vi "FlexMag - 24-03-2023.vi"() -> ()   [LabVIEW 2018] (continued)
    n6375 = Match Pattern(string=w11431, regular expression="¢") -> (after substring=w11429:string)  [unwired: 4 out]
    n6376 = String Length(string=w11429) -> (length=w11433:i32)
    n6377 = String Subset(string=w11429, length (rest)=1 ("length (rest)")) -> (substring=w11427:string)  [unwired: 1 out]
    n6378 = String To Byte Array(string=w11427) -> (unsigned byte array=w11426:u8[])
    n6379 = Not Equal To 0?(x=w11433) -> (x != 0?=w11432:bool)
    n6380 = Index Array(array=w11426, index=0) -> (element=w11424:u8)
    n6381 = String To Byte Array(string=w11401) -> (unsigned byte array=w11406:u8[])
    n6382 = Number To Boolean Array(number=w11424) -> (Boolean array=w11423:bool[])
    n6383 = case shown="True" w11432 {
      tunnel: [w11788 w11792] -> w11374
      tunnel: [w11787 w11791] -> w11373
      tunnel: w11421 -> [w11788 w11790]
      tunnel: w11420 -> [w11787 w11789]
      frame False {
      }
      frame True {
        n6384 = VISA Write(VISA resource name=w11790, write buffer="\u0006", error in (no error)=w11789) -> (VISA resource name out=w11792:refnum<visa-resource-name>, error out=w11791:errorcluster)  [unwired: 1 out]
      }
    }
    n6385 = for {
      tunnel: w11406 -> [w11776] mode=indexing
      shift-right: [w11774] -> w11404
      shift-left: 0 -> [w11775]
      n6386 = Exclusive Or(1:w11775, 2:w11776) -> (0:w11774:i32)
    }
    n6387 = Index Array(array=w11423, index=6) -> (element=→"RF 1 On":bool)
    n6388 = Build Array(w11404) -> (w11403:i32[])
    n6389 = Byte Array To String(unsigned byte array=w11403) -> (string=w11402:string)
    n6390 = Concatenate Strings(w11401, w11402) -> (w11400:string)
    n6391 = VISA Write(VISA resource name=w11374, write buffer=w11400, error in (no error)=w11373) -> (VISA resource name out=w11416:refnum<visa-resource-name>, error out=w11415:errorcluster)  [unwired: 1 out]
    n6392 = stacked-sequence {
      tunnel: [w11786] -> w11412
      tunnel: w11416 -> [w11786]
      tunnel: [w11785] -> w11411
      tunnel: w11415 -> [w11785]
      frame #0 {
        n6393 = Wait Until Next ms Multiple(millisecond multiple=u32 40) -> ()  [unwired: 1 out]
      }
    }
    n6394 = property class="Instr"(reference=w11412, error in=w11411) -> (reference out=w11418:refnum<visa-resource-name>, error out=w11417:errorcluster, "Serial Settings:Number of Bytes at Serial Port"=w11376:u32)
    n6395 = VISA Read(VISA resource name=w11418, byte count=w11376, error in (no error)=w11417) -> (VISA resource name out=w11410:refnum<visa-resource-name>, read buffer=w11413:string, error out=w11409:errorcluster)  [unwired: 1 out]
    n6396 = Match Pattern(string=w11413, regular expression="—") -> (after substring=w11407:string)  [unwired: 4 out]
    n6397 = String Length(string=w11407) -> (length=w11408:i32)
    n6398 = String To Byte Array(string=w11407) -> (unsigned byte array=w11379:u8[])
    n6399 = Not Equal To 0?(x=w11408) -> (x != 0?=w11375:bool)
    n6400 = Index Array(array=w11379, index=1) -> (element=w11395:u8)
    n6401 = Index Array(array=w11379, index=0) -> (element=w11392:u8)
    n6402 = Index Array(array=w11379, index=3) -> (element=w11390:u8)
    n6403 = Index Array(array=w11379, index=2) -> (element=w11389:u8)
    n6404 = To Unsigned Long Integer(number=w11395) -> (unsigned 32bit integer=w11394:u32)
    n6405 = To Unsigned Long Integer(number=w11392) -> (unsigned 32bit integer=w11391:u32)
    n6406 = To Unsigned Long Integer(number=w11390) -> (unsigned 32bit integer=w11387:u32)
    n6407 = To Unsigned Long Integer(number=w11389) -> (unsigned 32bit integer=w11388:u32)
    n6408 = case shown="True" w11375 {
      tunnel: w11410 -> [w11778 w11782]
      tunnel: w11409 -> [w11777 w11781]
      tunnel: [w11778 w11780] -> w11367
      tunnel: [w11777 w11779] -> w11366
      frame False {
      }
      frame True {
        n6409 = VISA Write(VISA resource name=w11782, write buffer="\u0006", error in (no error)=w11781) -> (VISA resource name out=w11780:refnum<visa-resource-name>, error out=w11779:errorcluster)  [unwired: 1 out]
      }
    }
    n6410 = local read "Forward Power"() -> (w11362:u32)
    n6411 = local read "Reflected Power"() -> (w11361:u32)
    n6412 = Multiply(x=w11394, y=256) -> (x*y=w11397:u32)
    n6413 = Multiply(x=256, y=w11387) -> (x*y=w11385:u32)
    n6414 = Add(x=w11397, y=w11391) -> (x+y=w11380:u32)
    n6415 = Add(x=w11385, y=w11388) -> (x+y=w11381:u32)
    n6416 = Subtract(x=w11362, y=w11361) -> (x-y=→"RF Net Power :":u32)
    n6417 = Divide(x=w11380, y=u32 10) -> (x/y=w11378:dbl)
    n6418 = Divide(x=w11381, y=u32 10) -> (x/y=w11377:dbl)
    n6419 = case shown="True" w11375 {
      tunnel: w11378 -> [_ w11773]
      tunnel: w11377 -> [_ w11772]
      frame False {
      }
      frame True {
        "Ramp Up Left Time:" <- w11773
        "Ramp Down Left Time:" <- w11772
      }
    }
    n6420 = VISA Write(VISA resource name=w11367, write buffer="\bキ", error in (no error)=w11366) -> (VISA resource name out=w11689:refnum<visa-resource-name>, error out=w11687:errorcluster)  [unwired: 1 out]
    n6421 = stacked-sequence {
      tunnel: [w11887] -> w11690
      tunnel: w11689 -> [w11887]
      tunnel: [w11886] -> w11688
      tunnel: w11687 -> [w11886]
      frame #0 {
        n6422 = Wait Until Next ms Multiple(millisecond multiple=u32 40) -> ()  [unwired: 1 out]
      }
    }
    n6423 = property class="Instr"(reference=w11690, error in=w11688) -> (reference out=w11705:refnum<visa-resource-name>, error out=w11704:errorcluster, "Serial Settings:Number of Bytes at Serial Port"=w11706:u32)
    n6424 = VISA Read(VISA resource name=w11705, byte count=w11706, error in (no error)=w11704) -> (VISA resource name out=w11686:refnum<visa-resource-name>, read buffer=w11691:string, error out=w11685:errorcluster)  [unwired: 1 out]
    n6425 = Match Pattern(string=w11691, regular expression="¥") -> (after substring=w11683:string)  [unwired: 4 out]
    n6426 = String Length(string=w11683) -> (length=w11684:i32)
    n6427 = String Subset(string=w11683, length (rest)=2 ("length (rest)")) -> (substring=w11701:string)  [unwired: 1 out]
    n6428 = Not Equal To 0?(x=w11684) -> (x != 0?=w11458:bool)
    n6429 = String To Byte Array(string=w11701) -> (unsigned byte array=w11699:u8[])
    n6430 = case shown="True" w11458 {
      tunnel: w11686 -> [w11880 w11884]
      tunnel: w11685 -> [w11879 w11883]
      tunnel: [w11880 w11882] -> w11661
      tunnel: [w11879 w11881] -> w11660
      frame False {
      }
      frame True {
        n6431 = VISA Write(VISA resource name=w11884, write buffer="\u0006", error in (no error)=w11883) -> (VISA resource name out=w11882:refnum<visa-resource-name>, error out=w11881:errorcluster)  [unwired: 1 out]
      }
    }
    n6432 = Index Array(array=w11699, index=1) -> (element=w11696:u8)
    n6433 = Index Array(array=w11699, index=0) -> (element=w11693:u8)
    n6434 = To Unsigned Long Integer(number=w11696) -> (unsigned 32bit integer=w11695:u32)
    n6435 = To Unsigned Long Integer(number=w11693) -> (unsigned 32bit integer=w11692:u32)
    n6436 = Multiply(x=256, y=w11695) -> (x*y=w11694:u32)
    n6437 = Add(x=w11694, y=w11692) -> (x+y=w11507:u32)
    n6438 = case shown="True" w11458 {
      tunnel: w11507 -> [_ w11817]
      frame False {
      }
      frame True {
        "Forward Power" <- w11817
      }
    }
    n6439 = VISA Write(VISA resource name=w11661, write buffer="\b¨ ", error in (no error)=w11660) -> (VISA resource name out=w11666:refnum<visa-resource-name>, error out=w11665:errorcluster)  [unwired: 1 out]
    n6440 = stacked-sequence {
      tunnel: [w11878] -> w11664
      tunnel: w11666 -> [w11878]
      tunnel: [w11877] -> w11663
      tunnel: w11665 -> [w11877]
      frame #0 {
        n6441 = Wait Until Next ms Multiple(millisecond multiple=u32 40) -> ()  [unwired: 1 out]
      }
    }
    n6442 = property class="Instr"(reference=w11664, error in=w11663) -> (reference out=w11682:refnum<visa-resource-name>, error out=w11680:errorcluster, "Serial Settings:Number of Bytes at Serial Port"=w11681:u32)
    n6443 = VISA Read(VISA resource name=w11682, byte count=w11681, error in (no error)=w11680) -> (VISA resource name out=w11659:refnum<visa-resource-name>, read buffer=w11679:string, error out=w11658:errorcluster)  [unwired: 1 out]
    n6444 = Match Pattern(string=w11679, regular expression="¨") -> (after substring=w11657:string)  [unwired: 4 out]
    n6445 = String Length(string=w11657) -> (length=w11656:i32)
    n6446 = String Subset(string=w11657, length (rest)=2 ("length (rest)")) -> (substring=w11676:string)  [unwired: 1 out]
    n6447 = Not Equal To 0?(x=w11656) -> (x != 0?=w11457:bool)
    n6448 = String To Byte Array(string=w11676) -> (unsigned byte array=w11674:u8[])
    n6449 = case shown="True" w11457 {
      tunnel: w11659 -> [w11870 w11874]
      tunnel: w11658 -> [w11869 w11873]
      tunnel: [w11870 w11872] -> w11620
      tunnel: [w11869 w11871] -> w11613
      frame False {
      }
      frame True {
        n6450 = VISA Write(VISA resource name=w11874, write buffer="\u0006", error in (no error)=w11873) -> (VISA resource name out=w11872:refnum<visa-resource-name>, error out=w11871:errorcluster)  [unwired: 1 out]
      }
    }
    n6451 = Index Array(array=w11674, index=1) -> (element=w11669:u8)
    n6452 = Index Array(array=w11674, index=0) -> (element=w11670:u8)
    n6453 = To Unsigned Long Integer(number=w11669) -> (unsigned 32bit integer=w11672:u32)
    n6454 = To Unsigned Long Integer(number=w11670) -> (unsigned 32bit integer=w11667:u32)
    n6455 = Multiply(x=256, y=w11672) -> (x*y=w11668:u32)
    n6456 = Add(x=w11668, y=w11667) -> (x+y=w11506:u32)
    n6457 = case shown="True" w11457 {
      tunnel: w11506 -> [_ w11816]
      frame False {
      }
      frame True {
        "RF Bias:" <- w11816
      }
    }
    n6458 = VISA Write(VISA resource name=w11620, write buffer="\b¯§", error in (no error)=w11613) -> (VISA resource name out=w11652:refnum<visa-resource-name>, error out=w11651:errorcluster)  [unwired: 1 out]
    n6459 = stacked-sequence {
      tunnel: [w11868] -> w11625
      tunnel: w11652 -> [w11868]
      tunnel: [w11867] -> w11624
      tunnel: w11651 -> [w11867]
      frame #0 {
        n6460 = Wait Until Next ms Multiple(millisecond multiple=u32 40) -> ()  [unwired: 1 out]
      }
    }
    n6461 = property class="Instr"(reference=w11625, error in=w11624) -> (reference out=w11654:refnum<visa-resource-name>, error out=w11653:errorcluster, "Serial Settings:Number of Bytes at Serial Port"=w11655:u32)
    n6462 = VISA Read(VISA resource name=w11654, byte count=w11655, error in (no error)=w11653) -> (VISA resource name out=w11619:refnum<visa-resource-name>, read buffer=w11626:string, error out=w11618:errorcluster)  [unwired: 1 out]
    n6463 = Match Pattern(string=w11626, regular expression="¯") -> (after substring=w11616:string)  [unwired: 4 out]
    n6464 = String Length(string=w11616) -> (length=w11617:i32)
    n6465 = String Subset(string=w11616, length (rest)=2 ("length (rest)")) -> (substring=w11643:string)  [unwired: 1 out]
    n6466 = String Subset(string=w11616, offset (0)=2, length (rest)=2 ("length (rest)")) -> (substring=w11638:string)
    n6467 = Not Equal To 0?(x=w11617) -> (x != 0?=w11456:bool)
    n6468 = String To Byte Array(string=w11643) -> (unsigned byte array=w11646:u8[])
    n6469 = String To Byte Array(string=w11638) -> (unsigned byte array=w11640:u8[])
    n6470 = case shown="True" w11456 {
      tunnel: [w11860 w11864] -> w11594
      tunnel: [w11859 w11863] -> w11593
      tunnel: w11619 -> [w11860 w11862]
      tunnel: w11618 -> [w11859 w11861]
      frame False {
      }
      frame True {
        n6471 = VISA Write(VISA resource name=w11862, write buffer="\u0006", error in (no error)=w11861) -> (VISA resource name out=w11864:refnum<visa-resource-name>, error out=w11863:errorcluster)  [unwired: 1 out]
      }
    }
    n6472 = Index Array(array=w11646, index=1) -> (element=w11637:u8)
    n6473 = Index Array(array=w11646, index=0) -> (element=w11634:u8)
    n6474 = Index Array(array=w11640, index=1) -> (element=w11632:u8)
    n6475 = Index Array(array=w11640, index=0) -> (element=w11631:u8)
    n6476 = To Unsigned Long Integer(number=w11637) -> (unsigned 32bit integer=w11636:u32)
    n6477 = To Unsigned Long Integer(number=w11634) -> (unsigned 32bit integer=w11633:u32)
    n6478 = To Unsigned Long Integer(number=w11632) -> (unsigned 32bit integer=w11629:u32)
    n6479 = To Unsigned Long Integer(number=w11631) -> (unsigned 32bit integer=w11630:u32)
    n6480 = Multiply(x=w11636, y=256) -> (x*y=w11644:u32)
    n6481 = Multiply(x=256, y=w11629) -> (x*y=w11627:u32)
    n6482 = Add(x=w11644, y=w11633) -> (x+y=w11614:u32)
    n6483 = Add(x=w11627, y=w11630) -> (x+y=w11615:u32)
    n6484 = case shown="True" w11456 {
      tunnel: u32 10 ("y") -> [_ w11815]
      tunnel: u32 10 ("y") -> [_ w11814]
      tunnel: w11615 -> [_ w11813]
      tunnel: w11614 -> [_ w11812]
      frame False {
      }
      frame True {
        n6485 = Divide(x=w11812, y=w11815) -> (x/y=→"CL Position:":dbl)
        n6486 = Divide(x=w11813, y=w11814) -> (x/y=→"CT Position:":dbl)
      }
    }
    n6487 = VISA Write(VISA resource name=w11594, write buffer="\bš’", error in (no error)=w11593) -> (VISA resource name out=w11609:refnum<visa-resource-name>, error out=w11608:errorcluster)  [unwired: 1 out]
    n6488 = stacked-sequence {
      tunnel: [w11858] -> w11596
      tunnel: w11609 -> [w11858]
      tunnel: [w11857] -> w11595
      tunnel: w11608 -> [w11857]
      frame #0 {
        n6489 = Wait Until Next ms Multiple(millisecond multiple=u32 40) -> ()  [unwired: 1 out]
      }
    }
    n6490 = property class="Instr"(reference=w11596, error in=w11595) -> (reference out=w11611:refnum<visa-resource-name>, error out=w11610:errorcluster, "Serial Settings:Number of Bytes at Serial Port"=w11612:u32)
    n6491 = VISA Read(VISA resource name=w11611, byte count=w11612, error in (no error)=w11610) -> (VISA resource name out=w11592:refnum<visa-resource-name>, read buffer=w11597:string, error out=w11591:errorcluster)  [unwired: 1 out]
    n6492 = Match Pattern(string=w11597, regular expression="\u0006\tš") -> (after substring=w11589:string)  [unwired: 4 out]
    n6493 = String Length(string=w11589) -> (length=w11590:i32)
    n6494 = String Subset(string=w11589, length (rest)=1 ("length (rest)")) -> (substring=w11598:string)  [unwired: 1 out]
    n6495 = Not Equal To 0?(x=w11590) -> (x != 0?=w11455:bool)
    n6496 = Match True/False String(2:"" ("false string"), 3:"\u0006" ("true string"), 4:w11598) -> (0:w11505:bool)  [unwired: 1 out]
    n6497 = Match True/False String(2:"" ("false string"), 3:"\b" ("true string"), 4:w11598) -> (0:w11504:bool)  [unwired: 1 out]
    n6498 = Match True/False String(2:"" ("false string"), 3:"\u0007" ("true string"), 4:w11598) -> (0:w11503:bool)  [unwired: 1 out]
    n6499 = case shown="True" w11455 {
      tunnel: [w11850 w11854] -> w11568
      tunnel: [w11849 w11851] -> w11567
      tunnel: w11592 -> [w11850 w11853]
      tunnel: w11591 -> [w11849 w11852]
      frame False {
      }
      frame True {
        n6500 = VISA Write(VISA resource name=w11853, write buffer="\u0006", error in (no error)=w11852) -> (VISA resource name out=w11854:refnum<visa-resource-name>, error out=w11851:errorcluster)  [unwired: 1 out]
      }
    }
    n6501 = case shown="True" w11455 {
      tunnel: w11505 -> [_ w11809]
      tunnel: w11504 -> [_ w11808]
      tunnel: w11503 -> [_ w11807]
      frame False {
      }
      frame True {
        "FORWARD   REGULATION" <- w11809
        "LOAD  REGULATION" <- w11807
        "DC BIAS REGULATION" <- w11808
      }
    }
    n6502 = VISA Write(VISA resource name=w11568, write buffer="\b惫", error in (no error)=w11567) -> (VISA resource name out=w11582:refnum<visa-resource-name>, error out=w11581:errorcluster)  [unwired: 1 out]
    n6503 = stacked-sequence {
      tunnel: [w11848] -> w11570
      tunnel: w11582 -> [w11848]
      tunnel: [w11847] -> w11569
      tunnel: w11581 -> [w11847]
      frame #0 {
        n6504 = Wait Until Next ms Multiple(millisecond multiple=u32 40) -> ()  [unwired: 1 out]
      }
    }
    n6505 = property class="Instr"(reference=w11570, error in=w11569) -> (reference out=w11584:refnum<visa-resource-name>, error out=w11583:errorcluster, "Serial Settings:Number of Bytes at Serial Port"=w11585:u32)
    n6506 = VISA Read(VISA resource name=w11584, byte count=w11585, error in (no error)=w11583) -> (VISA resource name out=w11566:refnum<visa-resource-name>, read buffer=w11571:string, error out=w11565:errorcluster)  [unwired: 1 out]
    n6507 = Match Pattern(string=w11571, regular expression="±") -> (after substring=w11563:string)  [unwired: 4 out]
    n6508 = String Subset(string=w11563) -> (substring=w11572:string)  [unwired: 2 out]
    n6509 = String Length(string=w11563) -> (length=w11564:i32)
    n6510 = Not Equal To 0?(x=w11564) -> (x != 0?=w11454:bool)
    n6511 = Match True/False String(2:"" ("false string"), 3:"\u0002" ("true string"), 4:w11572) -> (0:w11502:bool)  [unwired: 1 out]
    n6512 = Match True/False String(2:"" ("false string"), 3:"\u0000" ("true string"), 4:w11572) -> (0:w11501:bool)  [unwired: 1 out]
    n6513 = Match True/False String(2:"" ("false string"), 3:"\u0001" ("true string"), 4:w11572) -> (0:w11500:bool)  [unwired: 1 out]
    n6514 = case shown="True" w11454 {
      tunnel: [w11840 w11842] -> w11550
      tunnel: [w11839 w11841] -> w11549
      tunnel: w11566 -> [w11840 w11844]
      tunnel: w11565 -> [w11839 w11843]
      frame False {
      }
      frame True {
        n6515 = VISA Write(VISA resource name=w11844, write buffer="\u0006", error in (no error)=w11843) -> (VISA resource name out=w11842:refnum<visa-resource-name>, error out=w11841:errorcluster)  [unwired: 1 out]
      }
    }
    n6516 = case shown="True" w11454 {
      tunnel: w11502 -> [_ w11806]
      tunnel: w11501 -> [_ w11805]
      tunnel: w11500 -> [_ w11803]
      frame False {
      }
      frame True {
        n6517 = Not(x=w11805) -> (.not. x?=w11804:bool)
        n6518 = And(x=w11804, y=w11803) -> (x .and. y?=→"Pulsing ON/OFF :":bool)
        "INTERNAL PULSING" <- w11803
        "PULSING OFF" <- w11805
        "EXTERNAL PULSING" <- w11806
      }
    }
    n6519 = VISA Write(VISA resource name=w11550, write buffer="\b奶", error in (no error)=w11549) -> (VISA resource name out=w11559:refnum<visa-resource-name>, error out=w11558:errorcluster)  [unwired: 1 out]
    n6520 = stacked-sequence {
      tunnel: [w11838] -> w11552
      tunnel: w11559 -> [w11838]
      tunnel: [w11837] -> w11551
      tunnel: w11558 -> [w11837]
      frame #0 {
        n6521 = Wait Until Next ms Multiple(millisecond multiple=u32 40) -> ()  [unwired: 1 out]
      }
    }
    n6522 = property class="Instr"(reference=w11552, error in=w11551) -> (reference out=w11561:refnum<visa-resource-name>, error out=w11560:errorcluster, "Serial Settings:Number of Bytes at Serial Port"=w11562:u32)
    n6523 = VISA Read(VISA resource name=w11561, byte count=w11562, error in (no error)=w11560) -> (VISA resource name out=w11548:refnum<visa-resource-name>, read buffer=w11553:string, error out=w11547:errorcluster)  [unwired: 1 out]
    n6524 = Match Pattern(string=w11553, regular expression="Ä") -> (after substring=w11545:string)  [unwired: 4 out]
    n6525 = String To Byte Array(string=w11545) -> (unsigned byte array=w11555:u8[])
    n6526 = String Length(string=w11545) -> (length=w11453:i32)
    n6527 = Not Equal To 0?(x=w11453) -> (x != 0?=w11546:bool)
    n6528 = Index Array(array=w11555, index=0) -> (element=w11499:u8)
    n6529 = case shown="1" w11453 {
      tunnel: w11499 -> [_ w11801]
      frame 0, Default {
      }
      frame 1 {
        "duty cycle" <- w11801
      }
    }
    n6530 = case shown="True" w11546 {
      tunnel: [w11830 w11832] -> w11515
      tunnel: [w11829 w11831] -> w11514
      tunnel: w11548 -> [w11830 w11834]
      tunnel: w11547 -> [w11829 w11833]
      frame False {
      }
      frame True {
        n6531 = VISA Write(VISA resource name=w11834, write buffer="\u0006", error in (no error)=w11833) -> (VISA resource name out=w11832:refnum<visa-resource-name>, error out=w11831:errorcluster)  [unwired: 1 out]
      }
    }
    n6532 = VISA Write(VISA resource name=w11515, write buffer="\b辽", error in (no error)=w11514) -> (VISA resource name out=w11541:refnum<visa-resource-name>, error out=w11540:errorcluster)  [unwired: 1 out]
    n6533 = stacked-sequence {
      tunnel: [w11828] -> w11517
      tunnel: w11541 -> [w11828]
      tunnel: [w11827] -> w11516
      tunnel: w11540 -> [w11827]
      frame #0 {
        n6534 = Wait Until Next ms Multiple(millisecond multiple=u32 40) -> ()  [unwired: 1 out]
      }
    }
    n6535 = property class="Instr"(reference=w11517, error in=w11516) -> (reference out=w11543:refnum<visa-resource-name>, error out=w11542:errorcluster, "Serial Settings:Number of Bytes at Serial Port"=w11544:u32)
    n6536 = VISA Read(VISA resource name=w11543, byte count=w11544, error in (no error)=w11542) -> (VISA resource name out=w11513:refnum<visa-resource-name>, read buffer=w11518:string, error out=w11512:errorcluster)  [unwired: 1 out]
    n6537 = Match Pattern(string=w11518, regular expression="Á") -> (after substring=w11508:string)  [unwired: 4 out]
    n6538 = String To Byte Array(string=w11508) -> (unsigned byte array=w11531:u8[])
    n6539 = String Length(string=w11508) -> (length=w11452:i32)
    n6540 = Index Array(array=w11531, index=3) -> (element=w11523:u8)
    n6541 = Index Array(array=w11531, index=2) -> (element=w11526:u8)
    n6542 = Index Array(array=w11531, index=1) -> (element=w11535:u8)
    n6543 = Index Array(array=w11531, index=0) -> (element=w11533:u8)
    n6544 = Not Equal To 0?(x=w11452) -> (x != 0?=w11509:bool)
    n6545 = To Unsigned Long Integer(number=w11523) -> (unsigned 32bit integer=w11525:u32)
    n6546 = To Unsigned Long Integer(number=w11526) -> (unsigned 32bit integer=w11528:u32)
    n6547 = To Unsigned Long Integer(number=w11535) -> (unsigned 32bit integer=w11534:u32)
    n6548 = To Unsigned Long Integer(number=w11533) -> (unsigned 32bit integer=w11519:u32)
    n6549 = case shown="True" w11509 {
      tunnel: [w11820 w11822] -> w11511
      tunnel: [w11819 w11821] -> w11510
      tunnel: w11513 -> [w11820 w11824]
      tunnel: w11512 -> [w11819 w11823]
      frame False {
      }
      frame True {
        n6550 = VISA Write(VISA resource name=w11824, write buffer="\u0006", error in (no error)=w11823) -> (VISA resource name out=w11822:refnum<visa-resource-name>, error out=w11821:errorcluster)  [unwired: 1 out]
      }
    }
    n6551 = Multiply(x=256, y=w11525) -> (x*y=w11522:u32)
    n6552 = Multiply(x=256, y=w11528) -> (x*y=w11521:u32)
    n6553 = Multiply(x=256, y=w11534) -> (x*y=w11520:u32)
    n6554 = Compound Arithmetic op=ADD(w11522, w11521, w11520, w11519) -> (w11498:u32)
    n6555 = case shown="1" w11452 {
      tunnel: w11498 -> [_ w11800]
      frame 0, Default {
      }
      frame 1 {
        "Frequency" <- w11800
      }
    }
  }
  n6556 = property on="Tab Pressure Graph" class="TabCtl (strict)"("Visible"=FALSE) -> ()  [unwired: 2 in, 2 out]
  n6557 = while {
    i -> [w12239]
    stop <- FALSE stop-if-true
    n6558 = Get Date/Time String(want seconds? (F)=TRUE) -> (time string=w12257:string)  [unwired: 2 in, 1 out]
    "time string" <- w12257
    n6559 = local read "hour s"() -> (w12248:string)
    n6560 = local read "min s"() -> (w12247:string)
    n6561 = local read "sec s"() -> (w12246:string)
    n6562 = Match Pattern(string=w12257, regular expression=":") -> (before substring=→"hour s":string, after substring=w12255:string)  [unwired: 1 in, 2 out]
    n6563 = Match Pattern(string=w12255, regular expression=":") -> (before substring=→"min s":string, after substring=w12251:string)  [unwired: 1 in, 2 out]
    n6564 = call <vilib>:"Space Constant.vi"() -> ("String"=w12250:string)
    n6565 = Multiply(x=1000, y="graph sec") -> (x*y=w12242:dbl)
    n6566 = Decimal String To Number(string=w12248) -> (number=→"hour":i32)  [unwired: 2 in, 1 out]
    n6567 = Decimal String To Number(string=w12247) -> (number=→"min":i32)  [unwired: 2 in, 1 out]
    n6568 = Decimal String To Number(string=w12246) -> (number=→"sec":i32)  [unwired: 2 in, 1 out]
    n6569 = Build Array(FALSE, "show pressure graphs", "hide pressure graphs") -> (w12263:bool[])
    n6570 = Wait Until Next ms Multiple(millisecond multiple=w12242) -> ()  [unwired: 1 out]
    n6571 = Match Pattern(string=w12251, regular expression=w12250) -> (before substring=→"sec s":string)  [unwired: 1 in, 3 out]
    n6572 = Boolean Array To Number(Boolean array=w12263) -> (number=w12264:u32)
    n6573 = Mantissa & Exponent(0:w12264) -> (2:w12259:dbl)  [unwired: 1 out]
    n6574 = case shown="0, Default" w12259 {
      frame 0, Default {
      }
      frame 1 {
        n6575 = property on="Tab Pressure Graph" class="TabCtl (strict)"("Visible"=TRUE) -> ()  [unwired: 2 in, 2 out]
      }
      frame 2 {
        n6576 = property on="Tab Pressure Graph" class="TabCtl (strict)"("Visible"=FALSE) -> ()  [unwired: 2 in, 2 out]
      }
    }
    n6577 = local read "CH4_CC_DI"() -> (w12235:bool)
    n6578 = local read "CH3_CC_DI"() -> (w12236:bool)
    n6579 = local read "CH2_CC_DI"() -> (w12237:bool)
    n6580 = local read "CH1_CC_DI"() -> (w12238:bool)
    n6581 = case shown="False" w12235 {
      tunnel: [w12266 w12267] -> w12232
      frame False {
        n6582 = local read "ch4 ch pg mbar"() -> (w12266:dbl)
      }
      frame True {
        n6583 = local read "ch4 cc mbar"() -> (w12267:dbl)
      }
    }
    "CH 4 Pressure" <- w12232
    n6584 = case shown="False" w12236 {
      tunnel: [w12268 w12269] -> w12231
      frame False {
        n6585 = local read "ch3 ch pg mbar"() -> (w12268:dbl)
      }
      frame True {
        n6586 = local read "ch3 cc mbar"() -> (w12269:dbl)
      }
    }
    "CH 3 Pressure" <- w12231
    n6587 = case shown="False" w12237 {
      tunnel: [w12270 w12271] -> w12233
      frame False {
        n6588 = local read "ch2 ch pg mbar"() -> (w12270:dbl)
      }
      frame True {
        n6589 = local read "ch2 cc mbar"() -> (w12271:dbl)
      }
    }
    "CH 2 Pressure" <- w12233
    n6590 = case shown="False" w12238 {
      tunnel: [w12272 w12273] -> w12234
      frame False {
        n6591 = local read "ch1 ch pg mbar"() -> (w12272:dbl)
      }
      frame True {
        n6592 = local read "ch1 cc mbar"() -> (w12273:dbl)
      }
    }
    "CH 1 Pressure" <- w12234
    "iteration for graph" <- w12239
  }
  n6593 = while {
    i -> [w12277]
    stop <- FALSE stop-if-true
    n6594 = Greater?(x=w12277, y=u32 10 ("millisecond multiple")) -> (0:w12276:bool)
    n6595 = Wait Until Next ms Multiple(millisecond multiple=u32 1000) -> ()  [unwired: 1 out]
    n6596 = case shown="True" w12276 {
      frame False {
        n6597 = local read "ch2 ch pg torr"() -> (w12301:dbl)
        n6598 = local read "ch1 ch pg torr"() -> (w12304:dbl)
        n6599 = local read "ch3 ch pg torr"() -> (w12300:dbl)
        n6600 = local read "ch4 ch pg torr"() -> (w12293:dbl)
        n6601 = local read "ch2 ch pg torr"() -> (w12297:dbl)
        n6602 = local read "ch3 ch pg torr"() -> (w12296:dbl)
        n6603 = Less Or Equal?(x=w12301, y=50.0) -> (x <= y?=w12291:bool)
        n6604 = Less Or Equal?(x=w12304, y=50.0) -> (x <= y?=w12292:bool)
        n6605 = Less Or Equal?(x=w12300, y=50.0) -> (x <= y?=w12289:bool)
        n6606 = Less Or Equal?(x=w12293, y=50.0) -> (x <= y?=w12287:bool)
        n6607 = Less Or Equal?(x=w12297, y=50.0) -> (x <= y?=w12290:bool)
        n6608 = Less Or Equal?(x=w12296, y=50.0) -> (x <= y?=w12288:bool)
        n6609 = And(x=w12292, y=w12291) -> (x .and. y?=w12285:bool)
        n6610 = And(x=w12288, y=w12287) -> (x .and. y?=w12286:bool)
        n6611 = And(x=w12290, y=w12289) -> (x .and. y?=w12284:bool)
        n6612 = case shown="True" w12285 {
          tunnel: ["ATMOSPHERE" "VACUUM"] -> w12281
          frame False {
          }
          frame True {
          }
        }
        "ch1_2 vacuum level" <- w12281
        n6613 = case shown="True" w12284 {
          tunnel: ["ATMOSPHERE" "VACUUM"] -> w12283
          frame False {
          }
          frame True {
          }
        }
        "ch2_3 vacuum level" <- w12283
        n6614 = case shown="True" w12286 {
          tunnel: ["ATMOSPHERE" "VACUUM"] -> w12282
          frame False {
          }
          frame True {
          }
        }
        "ch3_4 vacuum level" <- w12282
      }
      frame True {
        n6615 = stacked-sequence {
          frame #0 {
            n6616 = local read "ch3_gv_bp_right_gui"() -> (w12334:bool)
            n6617 = local read "ch4_gv_bp_right_gui"() -> (w12324:bool)
            n6618 = local read "ch2_gv_bp_right_gui"() -> (w12344:bool)
            n6619 = local read "ch3_gv_bp_left_gui"() -> (w12325:bool)
            n6620 = local read "ch2_gv_bp_left_gui"() -> (w12335:bool)
            n6621 = local read "ch1_gv_bp_left_gui"() -> (w12345:bool)
            n6622 = feedback #181() -> (w12331:bool)  [unwired: 1 in]
            n6623 = feedback-in #181(w12334) -> ()
            n6624 = feedback #182() -> (w12328:bool)  [unwired: 1 in]
            n6625 = feedback-in #182(w12325) -> ()
            n6626 = feedback #183() -> (w12321:bool)  [unwired: 1 in]
            n6627 = feedback-in #183(w12324) -> ()
            n6628 = feedback #184() -> (w12338:bool)  [unwired: 1 in]
            n6629 = feedback-in #184(w12335) -> ()
            n6630 = feedback #185() -> (w12348:bool)  [unwired: 1 in]
            n6631 = feedback-in #185(w12345) -> ()
            n6632 = feedback #186() -> (w12341:bool)  [unwired: 1 in]
            n6633 = feedback-in #186(w12344) -> ()
            n6634 = Boolean To (0,1)(Boolean=w12334) -> (0, 1=w12330:i16)
            n6635 = Boolean To (0,1)(Boolean=w12325) -> (0, 1=w12329:i16)
            n6636 = Boolean To (0,1)(Boolean=w12324) -> (0, 1=w12320:i16)
            n6637 = Boolean To (0,1)(Boolean=w12335) -> (0, 1=w12339:i16)
            n6638 = Boolean To (0,1)(Boolean=w12331) -> (0, 1=w12332:i16)
            n6639 = Boolean To (0,1)(Boolean=w12328) -> (0, 1=w12327:i16)
            n6640 = Boolean To (0,1)(Boolean=w12321) -> (0, 1=w12322:i16)
            n6641 = Boolean To (0,1)(Boolean=w12345) -> (0, 1=w12349:i16)
            n6642 = Boolean To (0,1)(Boolean=w12344) -> (0, 1=w12340:i16)
            n6643 = Boolean To (0,1)(Boolean=w12338) -> (0, 1=w12337:i16)
            n6644 = Boolean To (0,1)(Boolean=w12348) -> (0, 1=w12347:i16)
            n6645 = Boolean To (0,1)(Boolean=w12341) -> (0, 1=w12342:i16)
            n6646 = Not Equal?(x=w12330, y=w12332) -> (x != y?=w12333:bool)
            n6647 = Not Equal?(x=w12329, y=w12327) -> (x != y?=w12326:bool)
            n6648 = Not Equal?(x=w12320, y=w12322) -> (x != y?=w12323:bool)
            n6649 = Not Equal?(x=w12339, y=w12337) -> (x != y?=w12336:bool)
            n6650 = Not Equal?(x=w12349, y=w12347) -> (x != y?=w12346:bool)
            n6651 = Not Equal?(x=w12340, y=w12342) -> (x != y?=w12343:bool)
            n6652 = case shown="True" w12333 {
              tunnel: w12334 -> [_ w12392]
              tunnel: [FALSE w12391] -> w12314
              frame False {
              }
              frame True {
                n6653 = case shown="True" w12392 {
                  tunnel: [FALSE TRUE] -> w12391
                  frame False {
                  }
                  frame True {
                  }
                }
              }
            }
            n6654 = case shown="True" w12326 {
              tunnel: w12325 -> [_ w12387]
              tunnel: [FALSE w12386] -> w12312
              frame False {
              }
              frame True {
                n6655 = case shown="True" w12387 {
                  tunnel: [FALSE TRUE] -> w12386
                  frame False {
                  }
                  frame True {
                  }
                }
              }
            }
            n6656 = case shown="True" w12323 {
              tunnel: w12324 -> [_ w12382]
              tunnel: [FALSE w12381] -> w12311
              frame False {
              }
              frame True {
                n6657 = case shown="True" w12382 {
                  tunnel: [FALSE TRUE] -> w12381
                  frame False {
                  }
                  frame True {
                  }
                }
              }
            }
            n6658 = case shown="True" w12336 {
              tunnel: w12335 -> [_ w12397]
              tunnel: [FALSE w12396] -> w12315
              frame False {
              }
              frame True {
                n6659 = case shown="True" w12397 {
                  tunnel: [FALSE TRUE] -> w12396
                  frame False {
                  }
                  frame True {
                  }
                }
              }
            }
            n6660 = case shown="True" w12346 {
              tunnel: w12345 -> [_ w12407]
              tunnel: [FALSE w12406] -> w12319
              frame False {
              }
              frame True {
                n6661 = case shown="True" w12407 {
                  tunnel: [FALSE TRUE] -> w12406
                  frame False {
                  }
                  frame True {
                  }
                }
              }
            }
            n6662 = case shown="True" w12343 {
              tunnel: w12344 -> [_ w12402]
              tunnel: [FALSE w12401] -> w12318
              frame False {
              }
              frame True {
                n6663 = case shown="True" w12402 {
                  tunnel: [FALSE TRUE] -> w12401
                  frame False {
                  }
                  frame True {
                  }
                }
              }
            }
            n6664 = Or(x=w12319, y=w12318) -> (x .or. y?=w12317:bool)
            n6665 = Or(x=w12315, y=w12314) -> (x .or. y?=w12316:bool)
            n6666 = Or(x=w12312, y=w12311) -> (x .or. y?=w12313:bool)
            n6667 = case shown="True" w12317 {
              frame False {
              }
              frame True {
                n6668 = local read "ch1 ch pg torr"() -> (w12377:dbl)
                n6669 = local read "ch2 ch pg torr"() -> (w12376:dbl)
                n6670 = Less?(x=w12377, y=0.5) -> (x < y?=w12373:bool)
                n6671 = Less?(x=w12376, y=0.5) -> (x < y?=w12372:bool)
                n6672 = And(x=w12373, y=w12372) -> (x .and. y?=w12370:bool)
                n6673 = case shown="False" w12370 {
                  tunnel: ["ATMOSPHERE" "VACUUM"] -> w12371
                  frame False {
                  }
                  frame True {
                  }
                }
                n6674 = local write "ch1_2 vacuum level"(w12371) -> ()
              }
            }
            n6675 = case shown="True" w12316 {
              frame False {
              }
              frame True {
                n6676 = local read "ch2 ch pg torr"() -> (w12367:dbl)
                n6677 = local read "ch3 ch pg torr"() -> (w12366:dbl)
                n6678 = Less?(x=w12367, y=0.5) -> (x < y?=w12363:bool)
                n6679 = Less?(x=w12366, y=0.5) -> (x < y?=w12362:bool)
                n6680 = And(x=w12363, y=w12362) -> (x .and. y?=w12361:bool)
                n6681 = case shown="True" w12361 {
                  tunnel: ["ATMOSPHERE" "VACUUM"] -> w12360
                  frame False {
                  }
                  frame True {
                  }
                }
                n6682 = local write "ch2_3 vacuum level"(w12360) -> ()
              }
            }
            n6683 = case shown="True" w12313 {
              frame False {
              }
              frame True {
                n6684 = local read "ch3 ch pg torr"() -> (w12357:dbl)
                n6685 = local read "ch4 ch pg torr"() -> (w12356:dbl)
                n6686 = Less?(x=w12357, y=0.5) -> (x < y?=w12353:bool)
                n6687 = Less?(x=w12356, y=0.5) -> (x < y?=w12352:bool)
                n6688 = And(x=w12353, y=w12352) -> (x .and. y?=w12351:bool)
                n6689 = case shown="False" w12351 {
                  tunnel: ["ATMOSPHERE" "VACUUM"] -> w12350
                  frame False {
                  }
                  frame True {
                  }
                }
                n6690 = local write "ch3_4 vacuum level"(w12350) -> ()
              }
            }
          }
          frame #1 {
            n6691 = local read "CH2_Trns_BP_Right_DI"() -> (w12414:bool)
            n6692 = local read "CH3_Trns_BP_Right_DI"() -> (w12413:bool)
            n6693 = local read "CH4_Trns_BP_Right_DI"() -> (w12410:bool)
            n6694 = local read "CH1_Trns_BP_Left_DI"() -> (w12415:bool)
            n6695 = local read "CH2_Trns_BP_Left_DI"() -> (w12412:bool)
            n6696 = local read "CH3_Trns_BP_Left_DI"() -> (w12411:bool)
            n6697 = case shown="True" w12415 {
              frame False {
              }
              frame True {
                n6698 = local read "ch1 ch pg torr"() -> (w12449:dbl)
                n6699 = Less?(x=w12449, y=0.5) -> (x < y?=w12446:bool)
                n6700 = case shown="True" w12446 {
                  tunnel: ["ATMOSPHERE" "VACUUM"] -> w12447
                  frame False {
                  }
                  frame True {
                  }
                }
                n6701 = local write "ch1_2 vacuum level"(w12447) -> ()
              }
            }
            n6702 = case shown="True" w12414 {
              frame False {
              }
              frame True {
                n6703 = local read "ch2 ch pg torr"() -> (w12443:dbl)
                n6704 = Less?(x=w12443, y=0.5) -> (x < y?=w12440:bool)
                n6705 = case shown="True" w12440 {
                  tunnel: ["ATMOSPHERE" "VACUUM"] -> w12441
                  frame False {
                  }
                  frame True {
                  }
                }
                n6706 = local write "ch1_2 vacuum level"(w12441) -> ()
              }
            }
            n6707 = case shown="True" w12412 {
              frame False {
              }
              frame True {
                n6708 = local read "ch2 ch pg torr"() -> (w12437:dbl)
                n6709 = Less?(x=w12437, y=0.5) -> (x < y?=w12434:bool)
                n6710 = case shown="True" w12434 {
                  tunnel: ["ATMOSPHERE" "VACUUM"] -> w12435
                  frame False {
                  }
                  frame True {
                  }
                }
                n6711 = local write "ch2_3 vacuum level"(w12435) -> ()
              }
            }
            n6712 = case shown="True" w12413 {
              frame False {
              }
              frame True {
                n6713 = local read "ch3 ch pg torr"() -> (w12431:dbl)
                n6714 = Less?(x=w12431, y=0.5) -> (x < y?=w12428:bool)
                n6715 = case shown="True" w12428 {
                  tunnel: ["ATMOSPHERE" "VACUUM"] -> w12429
                  frame False {
                  }
                  frame True {
                  }
                }
                n6716 = local write "ch2_3 vacuum level"(w12429) -> ()
              }
            }
            n6717 = case shown="True" w12411 {
              frame False {
              }
              frame True {
                n6718 = local read "ch3 ch pg torr"() -> (w12425:dbl)
                n6719 = Less?(x=w12425, y=0.5) -> (x < y?=w12422:bool)
                n6720 = case shown="True" w12422 {
                  tunnel: ["ATMOSPHERE" "VACUUM"] -> w12423
                  frame False {
                  }
                  frame True {
                  }
                }
                n6721 = local write "ch3_4 vacuum level"(w12423) -> ()
              }
            }
            n6722 = case shown="True" w12410 {
              frame False {
              }
              frame True {
                n6723 = local read "ch4 ch pg torr"() -> (w12419:dbl)
                n6724 = Less?(x=w12419, y=0.5) -> (x < y?=w12416:bool)
                n6725 = case shown="True" w12416 {
                  tunnel: ["ATMOSPHERE" "VACUUM"] -> w12417
                  frame False {
                  }
                  frame True {
                  }
                }
                n6726 = local write "ch3_4 vacuum level"(w12417) -> ()
              }
            }
          }
        }
      }
    }
  }
  n6727 = VISA Close(VISA resource name=w43, error in (no error)=w42) -> ()  [unwired: 1 out]
  n6728 = VISA Close(VISA resource name=w4, error in (no error)=w5) -> ()  [unwired: 1 out]
  n6729 = VISA Close(VISA resource name=w33, error in (no error)=w32) -> ()  [unwired: 1 out]
  n6730 = while {
    stop <- FALSE stop-if-true
    n6731 = local read "qr read statue"() -> (w12463:string)
    n6732 = Wait Until Next ms Multiple(millisecond multiple=u32 300) -> ()  [unwired: 1 out]
    n6733 = Equal?(x=w12463, y="0000" ("x")) -> (x = y?=w12493:bool)
    n6734 = Equal?(x=w12463, y="0001" ("x")) -> (x = y?=w12499:bool)
    n6735 = Equal?(x=w12463, y="0002" ("x")) -> (x = y?=w12486:bool)
    n6736 = Equal?(x=w12463, y="0003" ("x")) -> (x = y?=w12485:bool)
    n6737 = Equal?(x=w12463, y="0004" ("x")) -> (x = y?=w12484:bool)
    n6738 = Equal?(x=w12463, y="0005" ("x")) -> (x = y?=w12483:bool)
    n6739 = Equal?(x=w12463, y="0006" ("x")) -> (x = y?=w12481:bool)
    n6740 = Equal?(x=w12463, y="0007" ("x")) -> (x = y?=w12480:bool)
    n6741 = Equal?(x=w12463, y="0008" ("x")) -> (x = y?=w12479:bool)
    n6742 = Equal?(x=w12463, y="0009" ("x")) -> (x = y?=w12478:bool)
    n6743 = Equal?(x=w12463, y="0010" ("x")) -> (x = y?=w12462:bool)
    n6744 = Equal?(x=w12463, y="0011" ("x")) -> (x = y?=w12461:bool)
    n6745 = Equal?(x=w12463, y="0012" ("x")) -> (x = y?=w12460:bool)
    n6746 = Equal?(x=w12463, y="0013" ("x")) -> (x = y?=w12459:bool)
    n6747 = Equal?(x=w12463, y="0014" ("x")) -> (x = y?=w12458:bool)
    n6748 = Equal?(x=w12463, y="0015" ("x")) -> (x = y?=w12457:bool)
    n6749 = Equal?(x=w12463, y="0016" ("x")) -> (x = y?=w12456:bool)
    n6750 = Equal?(x=w12463, y="0017" ("x")) -> (x = y?=w12455:bool)
    n6751 = Equal?(x=w12463, y="0018" ("x")) -> (x = y?=w12454:bool)
    n6752 = Equal?(x=w12463, y="0019" ("x")) -> (x = y?=w12453:bool)
    n6753 = Equal?(x=w12463, y="0020" ("x")) -> (x = y?=w12452:bool)
    n6754 = Build Array(FALSE, w12493, w12499, w12486, w12485, w12484, w12483, w12481, w12480, w12479, w12478, w12462, w12461, w12460, w12459, w12458, w12457, w12456, w12455, w12454, w12453, w12452) -> (w12498:bool[])
    n6755 = Boolean Array To Number(Boolean array=w12498) -> (number=w12497:u32)
    n6756 = Mantissa & Exponent(0:w12497) -> (2:w12500:dbl)  [unwired: 1 out]
    n6757 = case shown="20" w12500 {
      frame 0, Default {
      }
      frame 1 {
        # "barcode 0"
        n6758 = stacked-sequence {
          frame #0 {
            n6759 = local read "forward roll"() -> (w12502:bool)
            n6760 = local read "back roll"() -> (w12501:bool)
            n6761 = case shown="False" w12502 {
              tunnel: w12501 -> [w12505 _]
              frame False {
                n6762 = case shown="True" w12505 {
                  frame False {
                  }
                  frame True {
                    n6763 = local write "backroll stop cmd"(TRUE ("backroll stop cmd")) -> ()
                  }
                }
              }
              frame True {
                n6764 = local write "forroll stop cmd"(TRUE ("forroll stop cmd")) -> ()
              }
            }
            n6765 = Wait (ms)(milliseconds to wait=u32 100) -> ()  [unwired: 1 out]
            n6766 = local write "QR off mode"(TRUE ("QR manual mode")) -> ()
          }
          frame #1 {
            n6767 = local read "qr wait second"() -> (w12508:u32)
            n6768 = Multiply(x=u32 1000 ("milliseconds to wait"), y=w12508) -> (x*y=w12509:u32)
            n6769 = Wait (ms)(milliseconds to wait=w12509) -> ()  [unwired: 1 out]
          }
          frame #2 {
            n6770 = local write "Interrupt DI"(TRUE ("Interrupt DI")) -> ()
            n6771 = Wait (ms)(milliseconds to wait=u32 100) -> ()  [unwired: 1 out]
          }
          frame #3 {
            n6772 = local read "forroll stop cmd"() -> (w12513:bool)
            n6773 = local read "backroll stop cmd"() -> (w12514:bool)
            n6774 = local read "step count"() -> (w12516:dbl)
            n6775 = Greater?(x=w12516, y=0.0) -> (0:w12517:bool)
            n6776 = case shown="True" w12513 {
              frame False {
              }
              frame True {
                n6777 = local write "forroll stop cmd"(FALSE ("backroll stop cmd")) -> ()
              }
            }
            n6778 = case shown="True" w12517 {
              frame False {
              }
              frame True {
                n6779 = local write "QR continuous mode"(TRUE ("QR continuous mode")) -> ()
              }
            }
            n6780 = case shown="True" w12514 {
              frame False {
              }
              frame True {
                n6781 = local write "backroll stop cmd"(FALSE ("backroll stop cmd")) -> ()
              }
            }
          }
        }
      }
      frame 2 {
        # "barcode 1"
        n6782 = stacked-sequence {
          frame #0 {
            n6783 = local read "forward roll"() -> (w12523:bool)
            n6784 = local read "step count 2"() -> (w12521:dbl)
            n6785 = local read "back roll"() -> (w12522:bool)
            n6786 = Wait (ms)(milliseconds to wait=u32 100) -> ()  [unwired: 1 out]
            n6787 = case shown="False" w12523 {
              tunnel: w12522 -> [w12526 _]
              tunnel: w12521 -> [_ w12529]
              frame False {
                n6788 = case shown="True" w12526 {
                  frame False {
                  }
                  frame True {
                    n6789 = stacked-sequence {
                      frame #0 {
                        n6790 = local write "current step"(1.0 ("current step")) -> ()
                      }
                      frame #1 {
                        n6791 = local write "step count"(1.0 ("y")) -> ()
                      }
                    }
                  }
                }
              }
              frame True {
                n6792 = stacked-sequence {
                  tunnel: w12529 -> [_ w12531]
                  frame #0 {
                    n6793 = local write "current step"(2.0 ("y")) -> ()
                  }
                  frame #1 {
                    n6794 = Subtract(x=w12531, y=1.0) -> (x-y=w12533:dbl)
                    n6795 = local write "step count"(w12533) -> ()
                  }
                }
              }
            }
            n6796 = local write "QR off mode"(TRUE ("QR manual mode")) -> ()
          }
          frame #1 {
            n6797 = local read "qr wait second"() -> (w12534:u32)
            n6798 = Multiply(x=u32 1000 ("milliseconds to wait"), y=w12534) -> (x*y=w12535:u32)
            n6799 = Wait (ms)(milliseconds to wait=w12535) -> ()  [unwired: 1 out]
          }
          frame #2 {
            n6800 = disable-structure shown="Disabled" {
              frame Disabled {
                n6801 = local write "Interrupt DI"(TRUE ("Interrupt DI")) -> ()
                n6802 = Wait (ms)(milliseconds to wait=u32 100) -> ()  [unwired: 1 out]
              }
              frame Enabled {
              }
            }
          }
          frame #3 {
            n6803 = local read "step count"() -> (w12540:dbl)
            n6804 = Greater?(x=w12540, y=0.0) -> (0:w12541:bool)
            n6805 = case shown="True" w12541 {
              frame False {
              }
              frame True {
                n6806 = local write "QR continuous mode"(TRUE ("QR continuous mode")) -> ()
              }
            }
          }
        }
      }
      frame 3 {
        # "barcode 2"
        n6807 = stacked-sequence {
          frame #0 {
            n6808 = local read "forward roll"() -> (w12545:bool)
            n6809 = local read "step count 2"() -> (w12543:dbl)
            n6810 = local read "back roll"() -> (w12544:bool)
            n6811 = Wait (ms)(milliseconds to wait=u32 100) -> ()  [unwired: 1 out]
            n6812 = case shown="True" w12545 {
              tunnel: w12544 -> [w12548 _]
              tunnel: w12543 -> [_ w12551]
              frame False {
                n6813 = case shown="True" w12548 {
                  frame False {
                  }
                  frame True {
                    n6814 = stacked-sequence {
                      frame #0 {
                        n6815 = local write "current step"(2.0 ("current step")) -> ()
                      }
                      frame #1 {
                        n6816 = local write "step count"(2.0 ("y")) -> ()
                      }
                    }
                  }
                }
              }
              frame True {
                n6817 = stacked-sequence {
                  tunnel: w12551 -> [_ w12553]
                  frame #0 {
                    n6818 = local write "current step"(3.0 ("y")) -> ()
                  }
                  frame #1 {
                    n6819 = Subtract(x=w12553, y=2.0) -> (x-y=w12555:dbl)
                    n6820 = local write "step count"(w12555) -> ()
                  }
                }
              }
            }
            n6821 = local write "QR off mode"(TRUE ("QR manual mode")) -> ()
          }
          frame #1 {
            n6822 = local read "qr wait second"() -> (w12556:u32)
            n6823 = Multiply(x=u32 1000 ("milliseconds to wait"), y=w12556) -> (x*y=w12557:u32)
            n6824 = Wait (ms)(milliseconds to wait=w12557) -> ()  [unwired: 1 out]
          }
          frame #2 {
            n6825 = disable-structure shown="Disabled" {
              frame Disabled {
                n6826 = local write "Interrupt DI"(TRUE ("Interrupt DI")) -> ()
                n6827 = Wait (ms)(milliseconds to wait=u32 100) -> ()  [unwired: 1 out]
              }
              frame Enabled {
              }
            }
          }
          frame #3 {
            n6828 = local read "step count"() -> (w12562:dbl)
            n6829 = Greater?(x=w12562, y=0.0) -> (0:w12563:bool)
            n6830 = case shown="True" w12563 {
              frame False {
              }
              frame True {
                n6831 = local write "QR continuous mode"(TRUE ("QR continuous mode")) -> ()
              }
            }
          }
        }
      }
      frame 4 {
        # "barcode 3"
        n6832 = stacked-sequence {
          frame #0 {
            n6833 = local read "forward roll"() -> (w12567:bool)
            n6834 = local read "step count 2"() -> (w12565:dbl)
            n6835 = local read "back roll"() -> (w12566:bool)
            n6836 = Wait (ms)(milliseconds to wait=u32 100) -> ()  [unwired: 1 out]
            n6837 = case shown="False" w12567 {
              tunnel: w12566 -> [w12570 _]
              tunnel: w12565 -> [_ w12573]
              frame False {
                n6838 = case shown="True" w12570 {
                  frame False {
                  }
                  frame True {
                    n6839 = stacked-sequence {
                      frame #0 {
                        n6840 = local write "current step"(3.0 ("current step")) -> ()
                      }
                      frame #1 {
                        n6841 = local write "step count"(3.0 ("y")) -> ()
                      }
                    }
                  }
                }
              }
              frame True {
                n6842 = stacked-sequence {
                  tunnel: w12573 -> [_ w12576]
                  frame #0 {
                    n6843 = local write "current step"(4.0 ("y")) -> ()
                  }
                  frame #1 {
                    n6844 = Subtract(x=w12576, y=3.0) -> (x-y=w12577:dbl)
                    n6845 = local write "step count"(w12577) -> ()
                  }
                }
              }
            }
            n6846 = local write "QR off mode"(TRUE ("QR manual mode")) -> ()
          }
          frame #1 {
            n6847 = local read "qr wait second"() -> (w12578:u32)
            n6848 = Multiply(x=u32 1000 ("milliseconds to wait"), y=w12578) -> (x*y=w12579:u32)
            n6849 = Wait (ms)(milliseconds to wait=w12579) -> ()  [unwired: 1 out]
          }
          frame #2 {
            n6850 = disable-structure shown="Disabled" {
              frame Disabled {
                n6851 = local write "Interrupt DI"(TRUE ("Interrupt DI")) -> ()
                n6852 = Wait (ms)(milliseconds to wait=u32 100) -> ()  [unwired: 1 out]
              }
              frame Enabled {
              }
            }
          }
          frame #3 {
            n6853 = local read "step count"() -> (w12584:dbl)
            n6854 = Greater?(x=w12584, y=0.0) -> (0:w12585:bool)
            n6855 = case shown="True" w12585 {
              frame False {
              }
              frame True {
                n6856 = local write "QR continuous mode"(TRUE ("QR continuous mode")) -> ()
              }
            }
          }
        }
      }
      frame 5 {
        # "barcode 4"
        n6857 = stacked-sequence {
          frame #0 {
            n6858 = local read "forward roll"() -> (w12589:bool)
            n6859 = local read "step count 2"() -> (w12587:dbl)
            n6860 = local read "back roll"() -> (w12588:bool)
            n6861 = Wait (ms)(milliseconds to wait=u32 100) -> ()  [unwired: 1 out]
            n6862 = case shown="False" w12589 {
              tunnel: w12588 -> [w12592 _]
              tunnel: w12587 -> [_ w12595]
              frame False {
                n6863 = case shown="True" w12592 {
                  frame False {
                  }
                  frame True {
                    n6864 = stacked-sequence {
                      frame #0 {
                        n6865 = local write "current step"(4.0 ("current step")) -> ()
                      }
                      frame #1 {
                        n6866 = local write "step count"(4.0 ("y")) -> ()
                      }
                    }
                  }
                }
              }
              frame True {
                n6867 = stacked-sequence {
                  tunnel: w12595 -> [_ w12598]
                  frame #0 {
                    n6868 = local write "current step"(5.0 ("y")) -> ()
                  }
                  frame #1 {
                    n6869 = Subtract(x=w12598, y=4.0) -> (x-y=w12599:dbl)
                    n6870 = local write "step count"(w12599) -> ()
                  }
                }
              }
            }
            n6871 = local write "QR off mode"(TRUE ("QR manual mode")) -> ()
          }
          frame #1 {
            n6872 = local read "qr wait second"() -> (w12600:u32)
            n6873 = Multiply(x=u32 1000 ("milliseconds to wait"), y=w12600) -> (x*y=w12601:u32)
            n6874 = Wait (ms)(milliseconds to wait=w12601) -> ()  [unwired: 1 out]
          }
          frame #2 {
            n6875 = disable-structure shown="Disabled" {
              frame Disabled {
                n6876 = local write "Interrupt DI"(TRUE ("Interrupt DI")) -> ()
                n6877 = Wait (ms)(milliseconds to wait=u32 100) -> ()  [unwired: 1 out]
              }
              frame Enabled {
              }
            }
          }
          frame #3 {
            n6878 = local read "step count"() -> (w12606:dbl)
            n6879 = Greater?(x=w12606, y=0.0) -> (0:w12607:bool)
            n6880 = case shown="True" w12607 {
              frame False {
              }
              frame True {
                n6881 = local write "QR continuous mode"(TRUE ("QR continuous mode")) -> ()
              }
            }
          }
        }
      }
      frame 6 {
        # "barcode 5"
        n6882 = stacked-sequence {
          frame #0 {
            n6883 = local read "forward roll"() -> (w12611:bool)
            n6884 = local read "step count 2"() -> (w12609:dbl)
            n6885 = local read "back roll"() -> (w12610:bool)
            n6886 = Wait (ms)(milliseconds to wait=u32 100) -> ()  [unwired: 1 out]
            n6887 = case shown="False" w12611 {
              tunnel: w12610 -> [w12614 _]
              tunnel: w12609 -> [_ w12617]
              frame False {
                n6888 = case shown="True" w12614 {
                  frame False {
                  }
                  frame True {
                    n6889 = stacked-sequence {
                      frame #0 {
                        n6890 = local write "current step"(5.0 ("current step")) -> ()
                      }
                      frame #1 {
                        n6891 = local write "step count"(5.0 ("y")) -> ()
                      }
                    }
                  }